vi "Main.vi"() -> ()   [LabVIEW 2015] (continued)
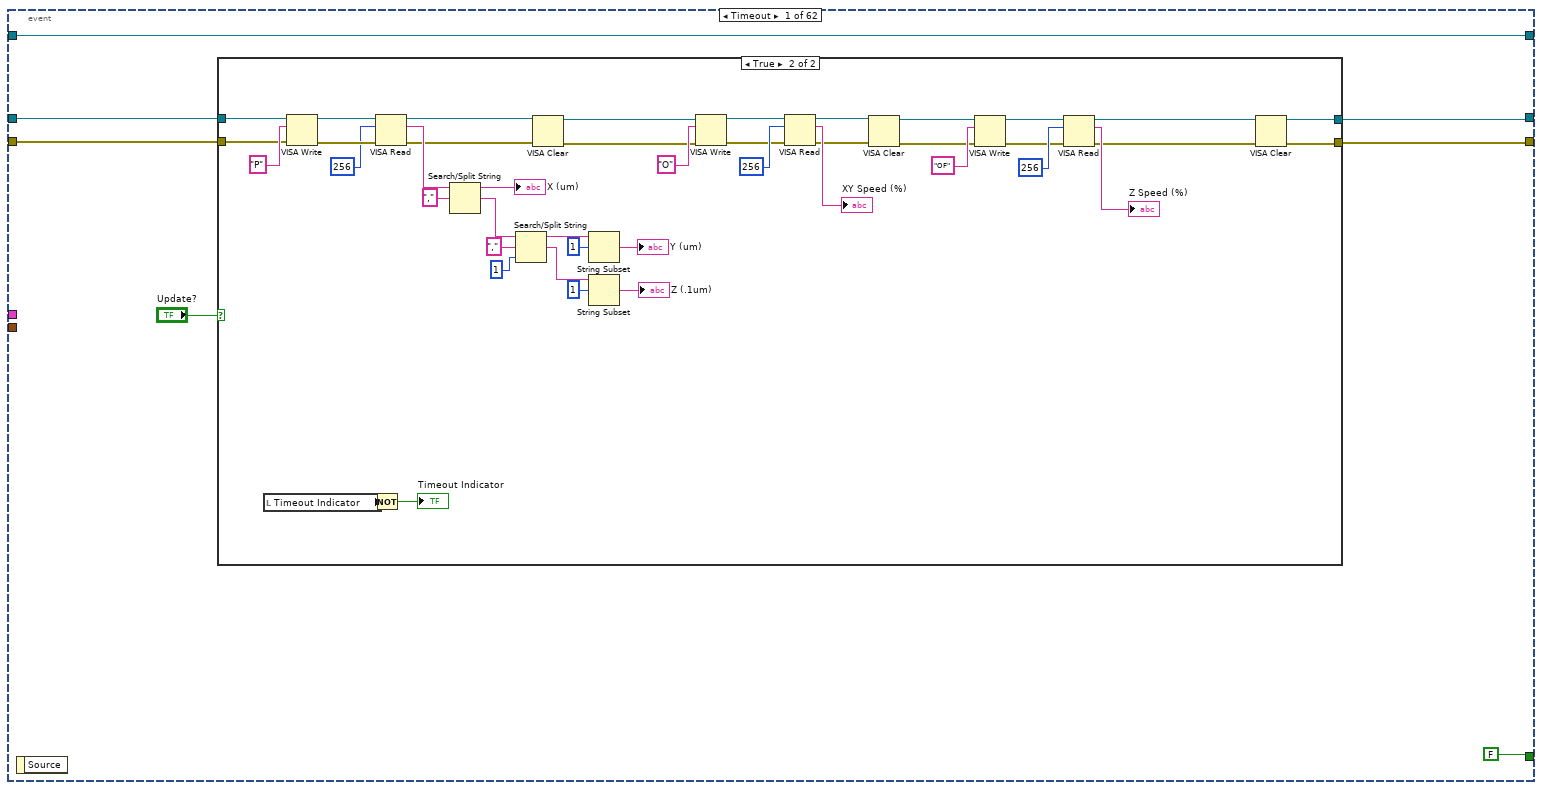
[diagram p3: hidden frame]
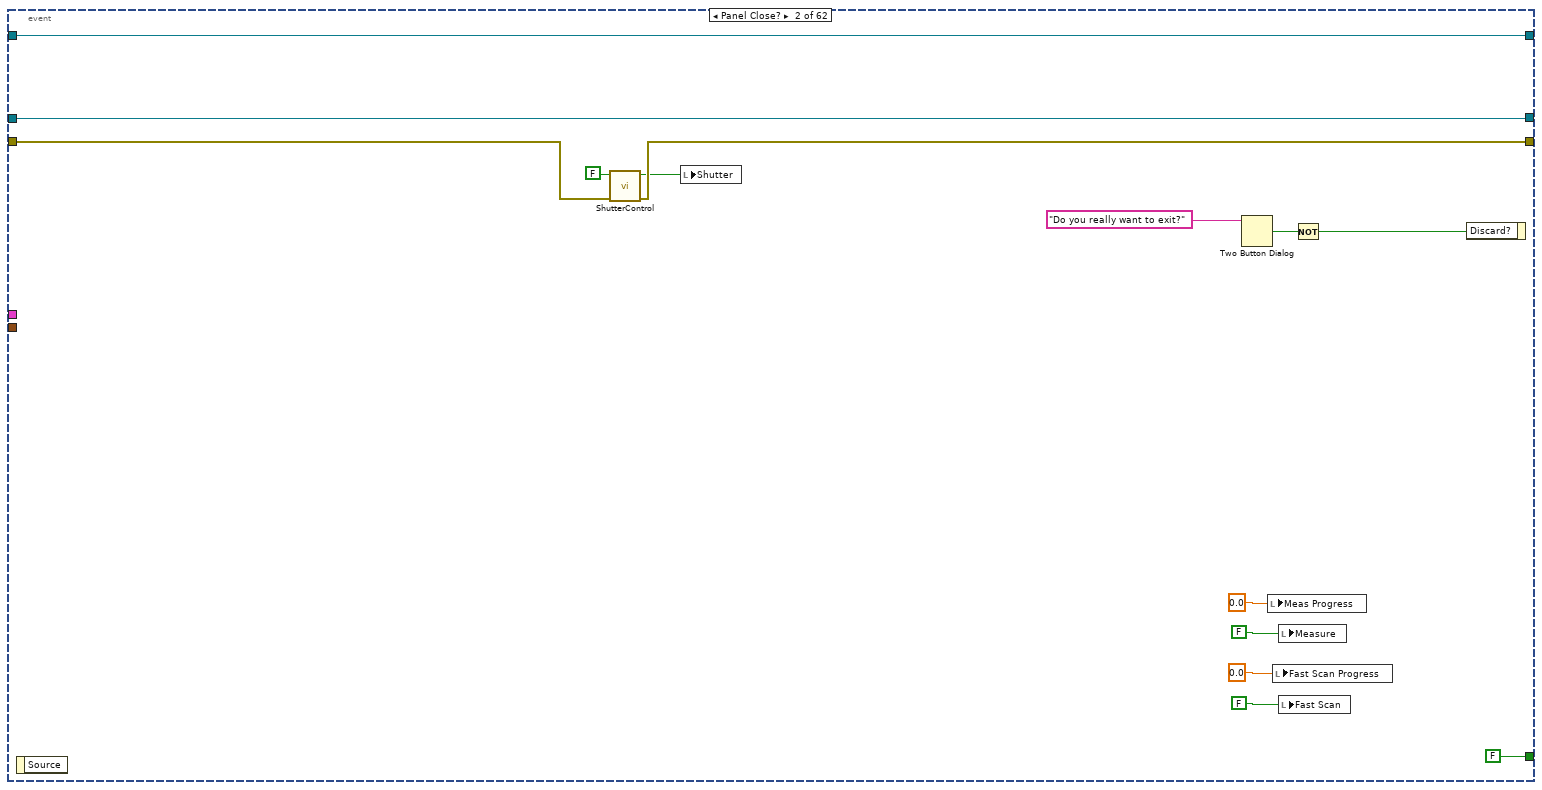
[diagram p5: hidden frame]
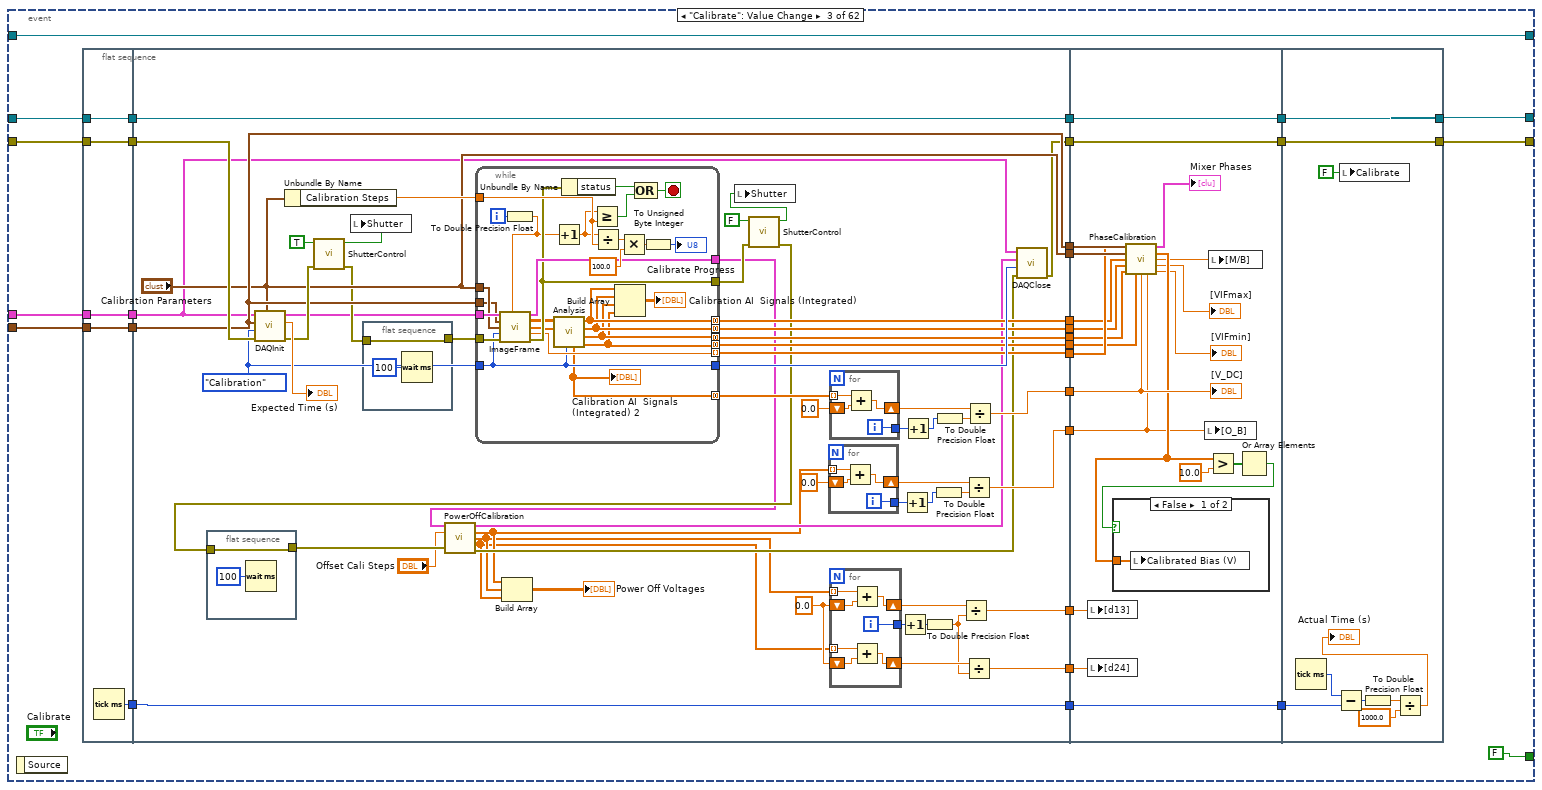
[diagram p6: hidden frame]
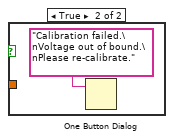
[diagram p7: hidden frame]
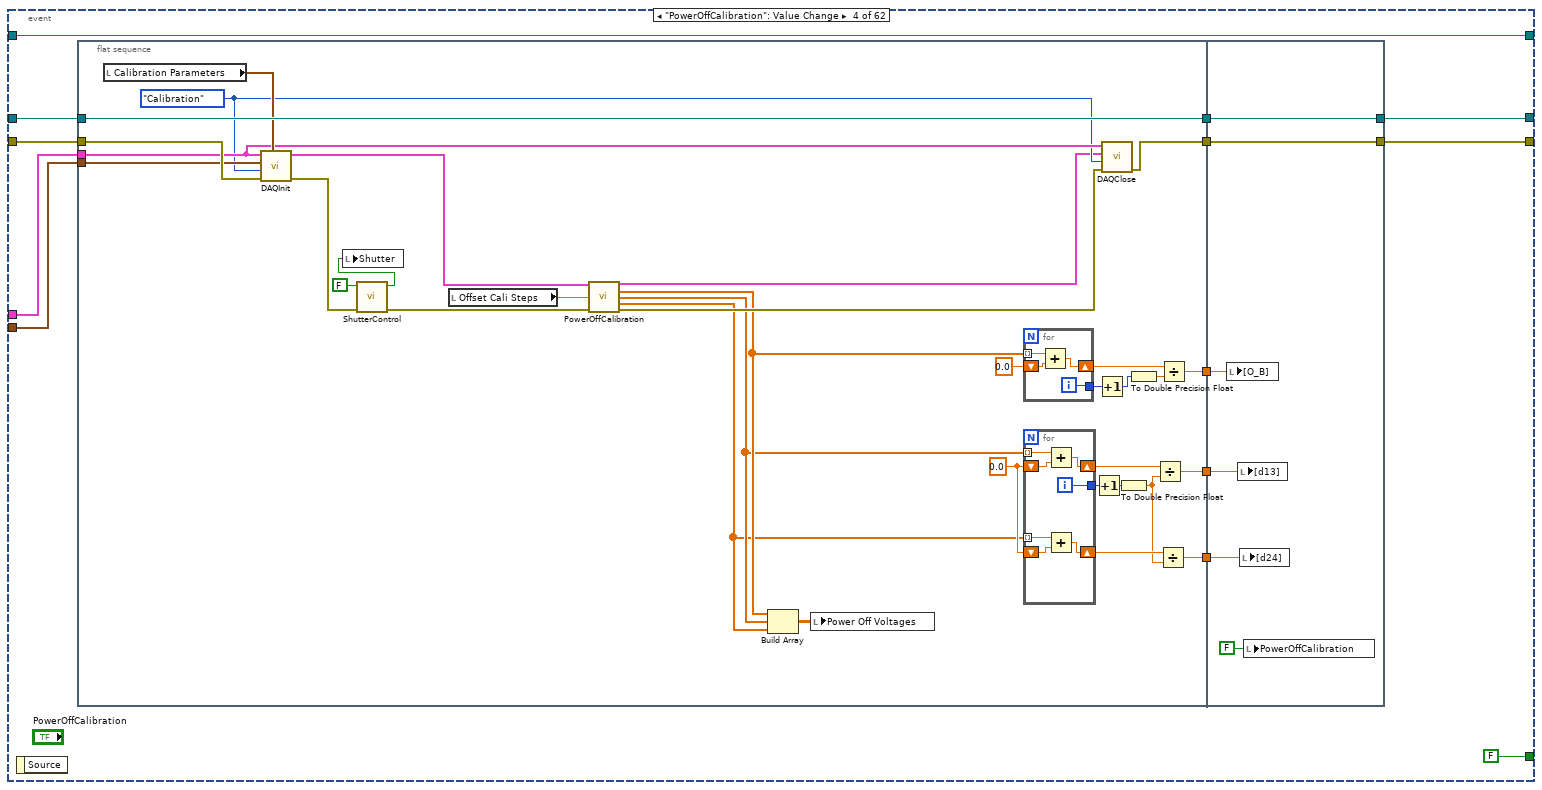
[diagram p8: hidden frame]
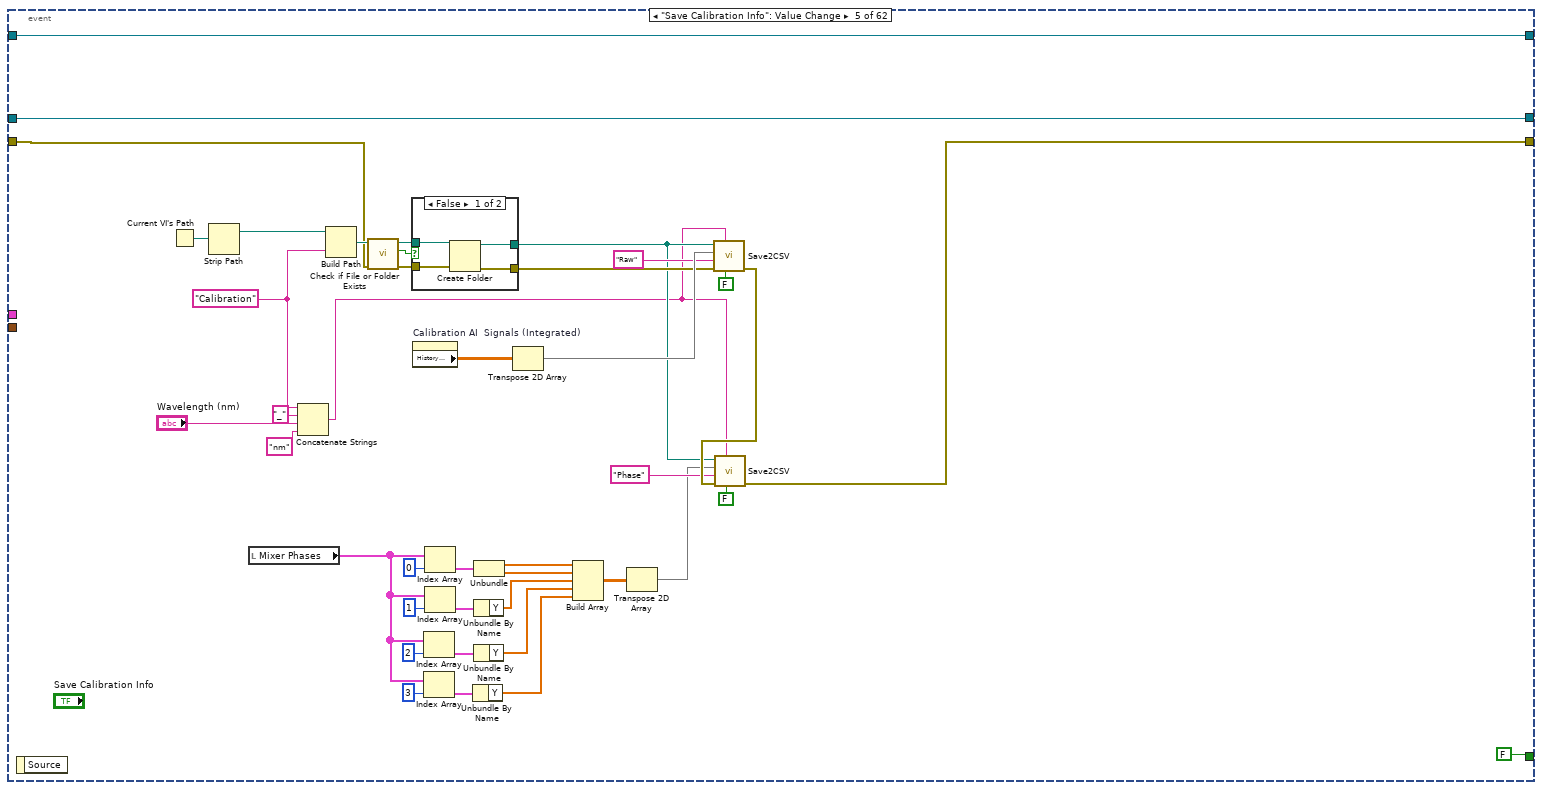
[diagram p9: hidden frame]
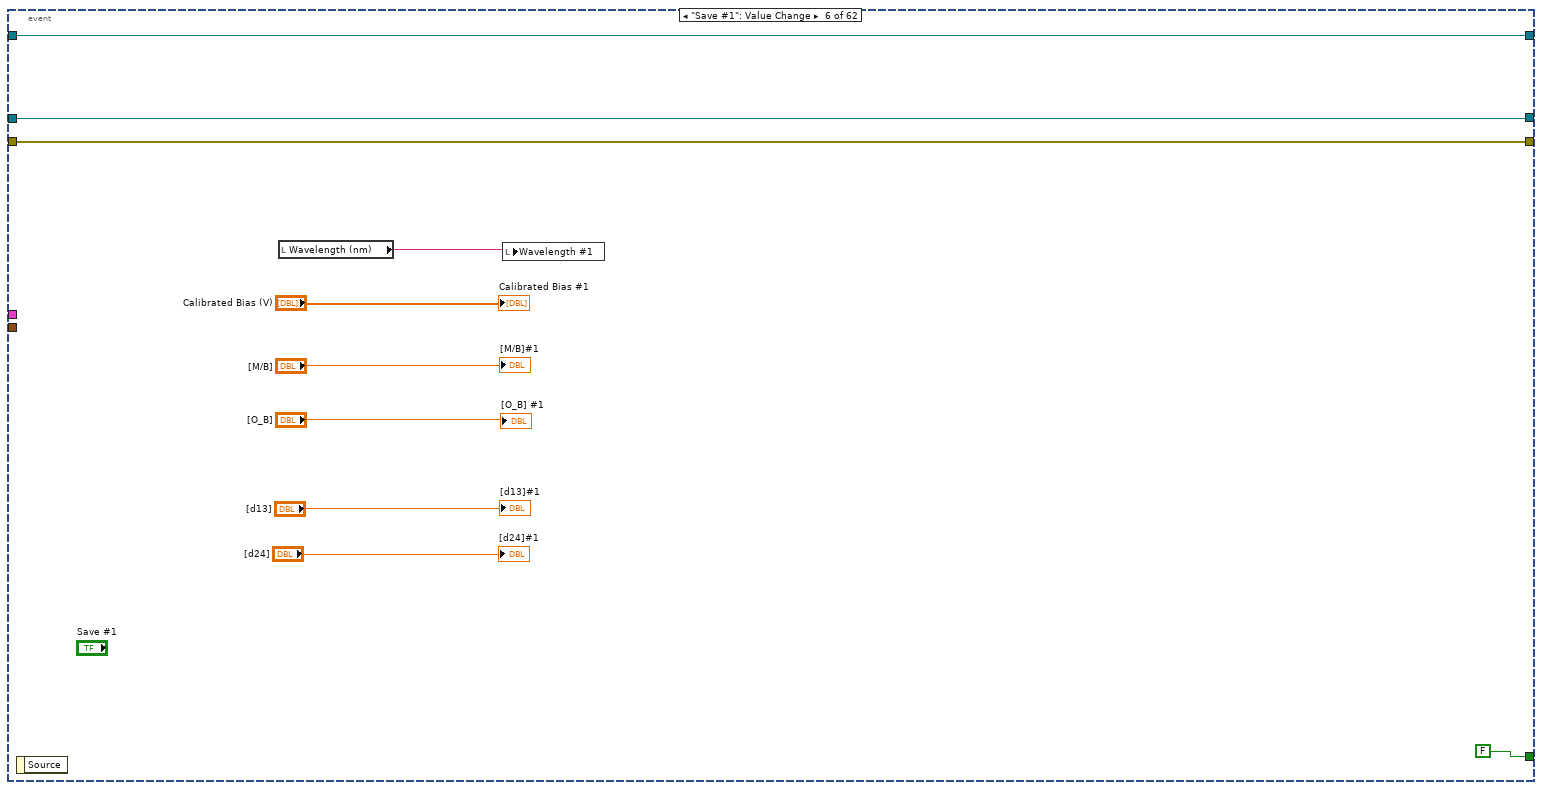
[diagram p11: hidden frame]
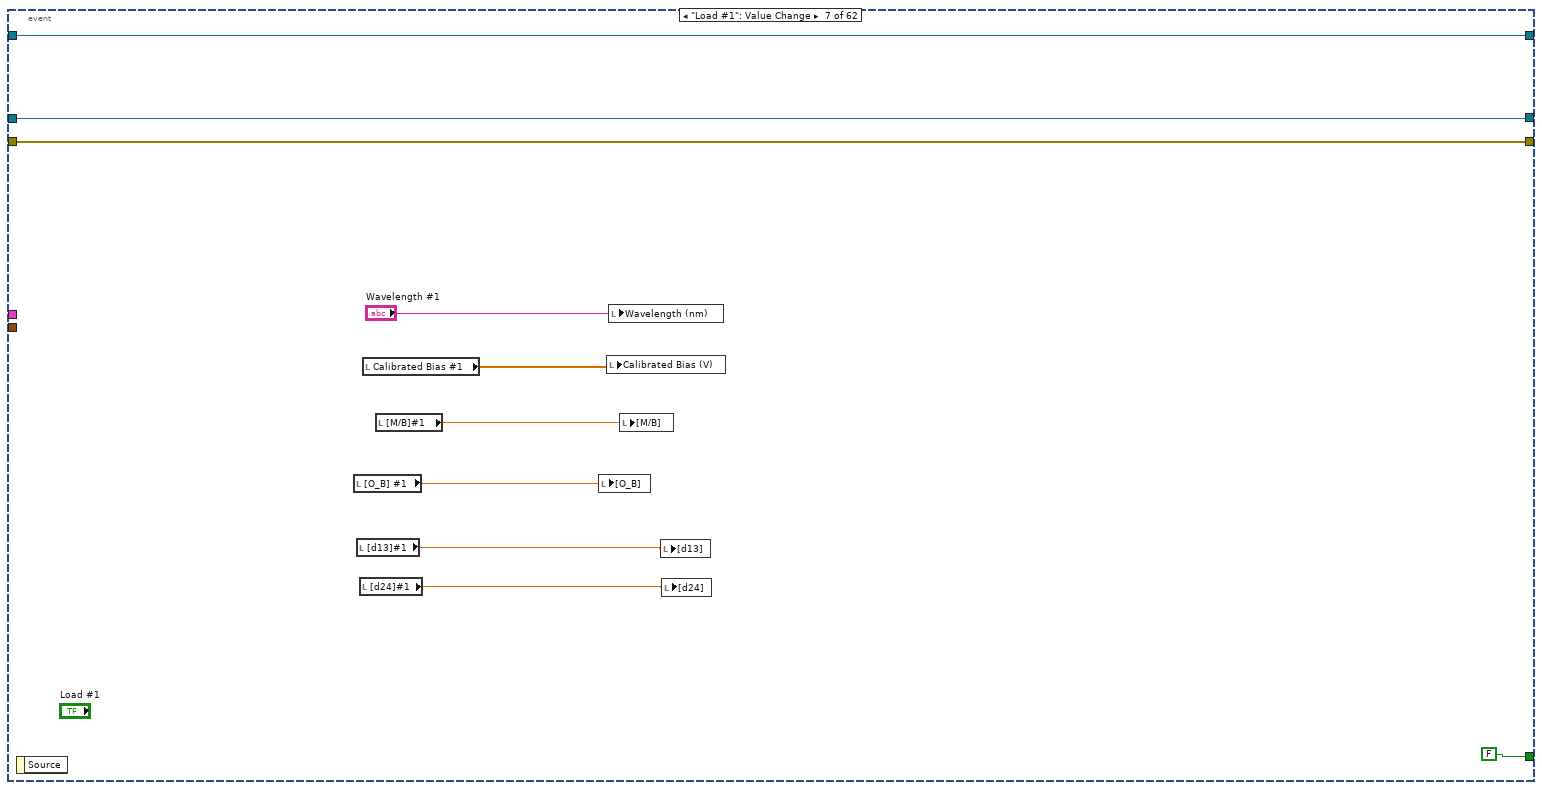
[diagram p12: hidden frame]
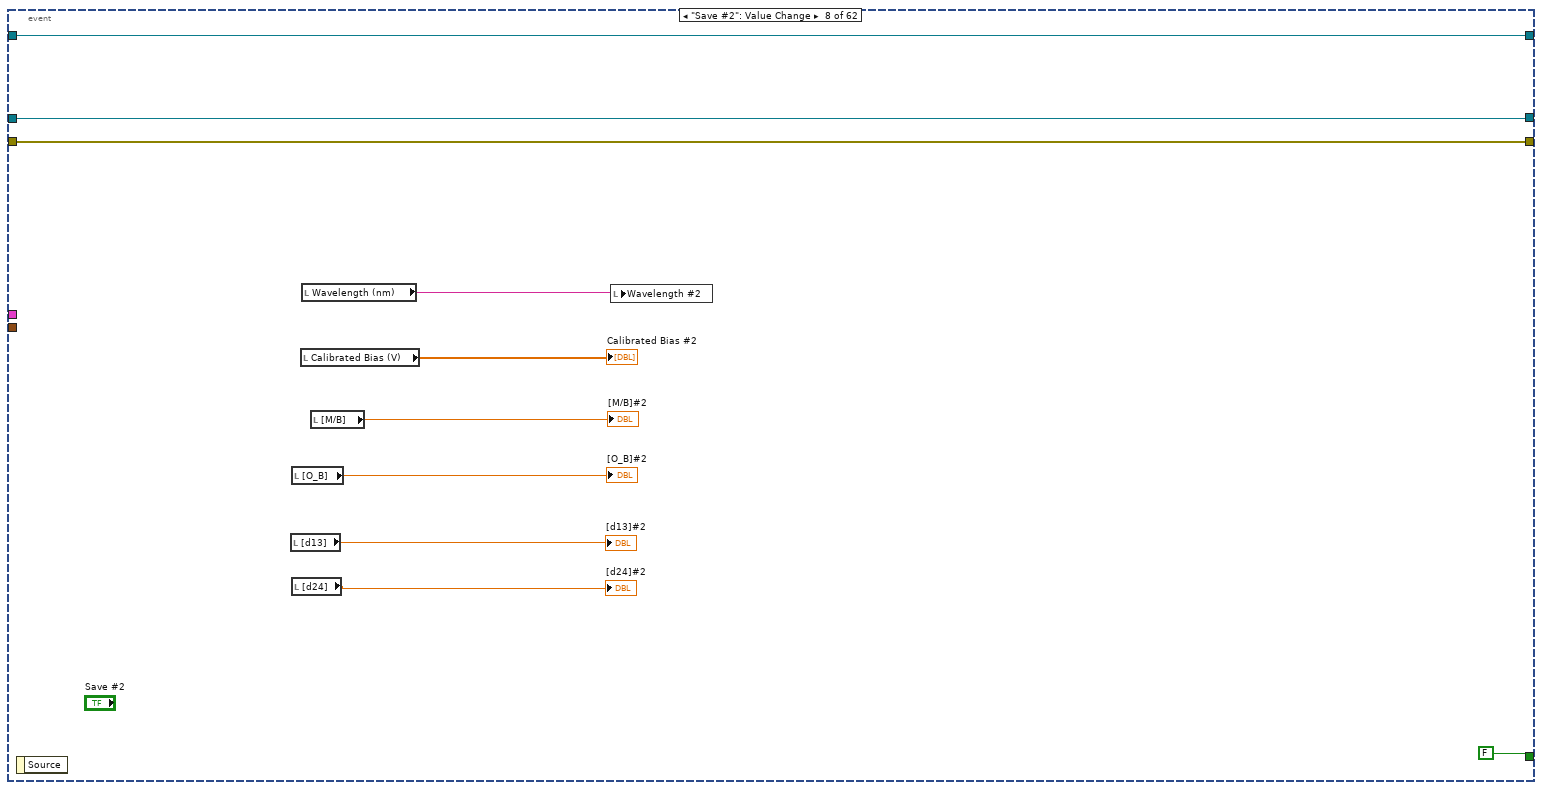
[diagram p13: hidden frame]
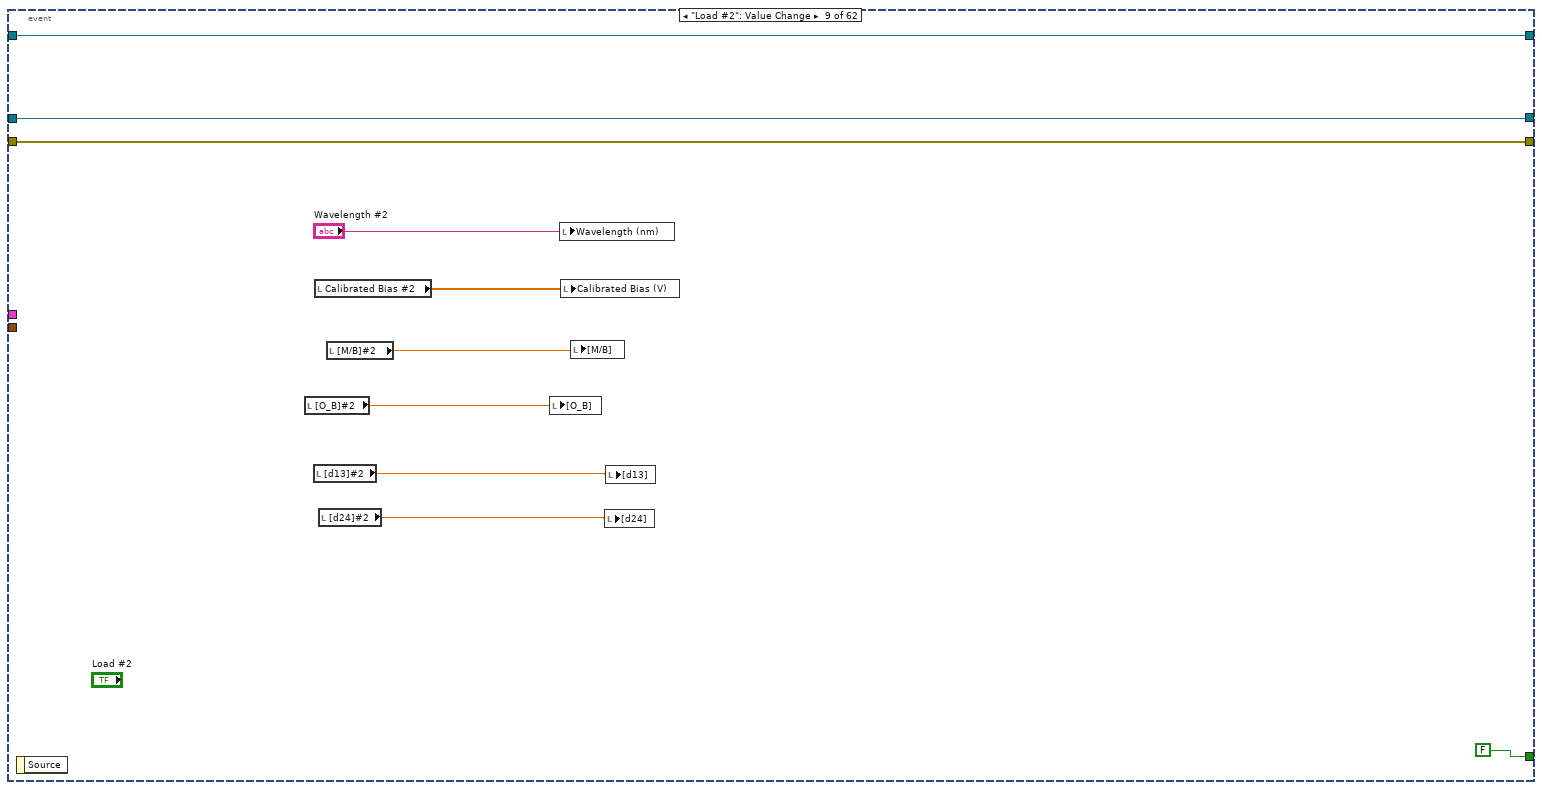
[diagram p14: hidden frame]
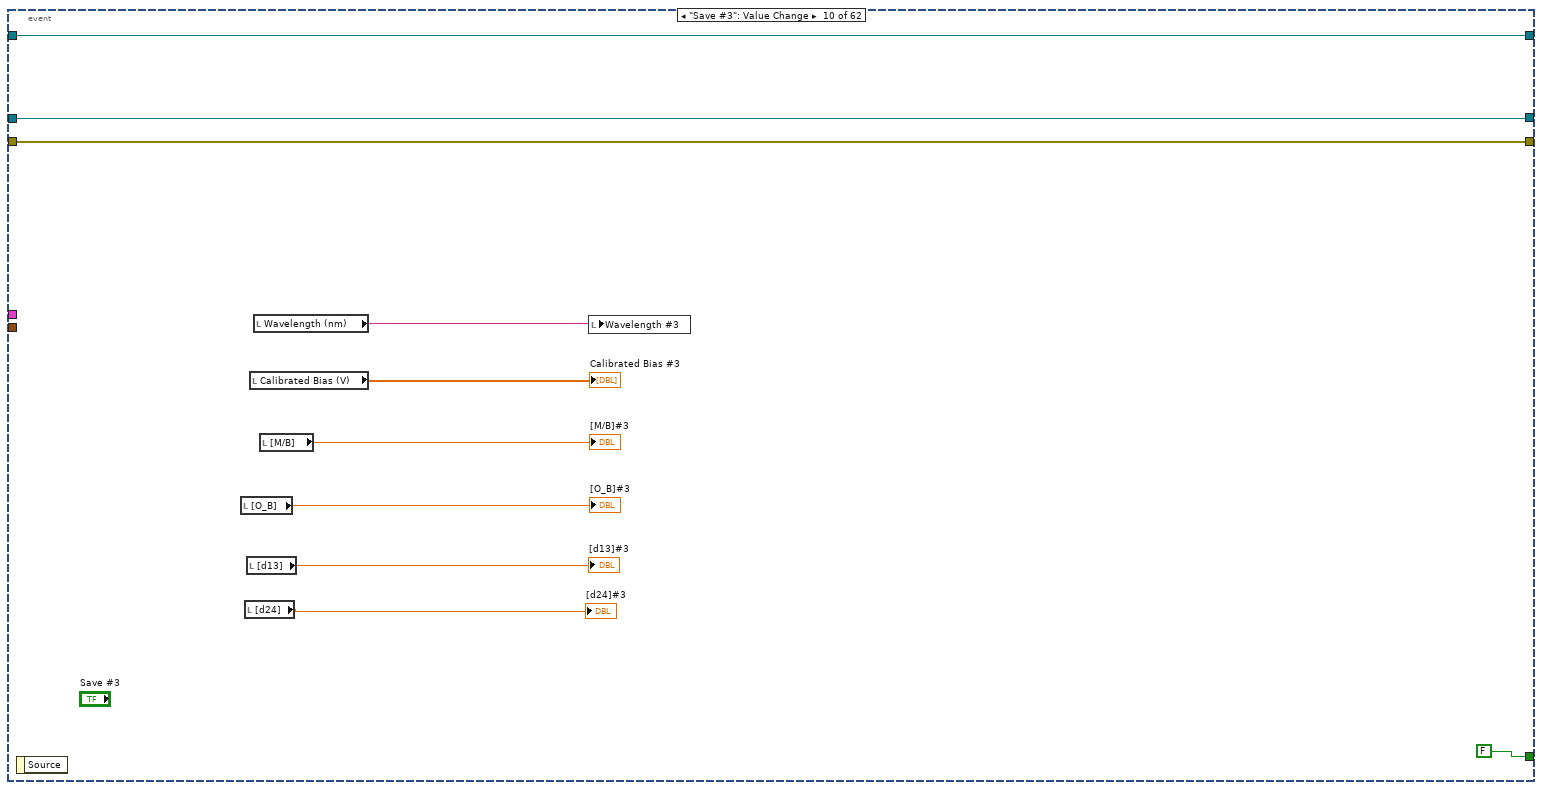
[diagram p15: hidden frame]
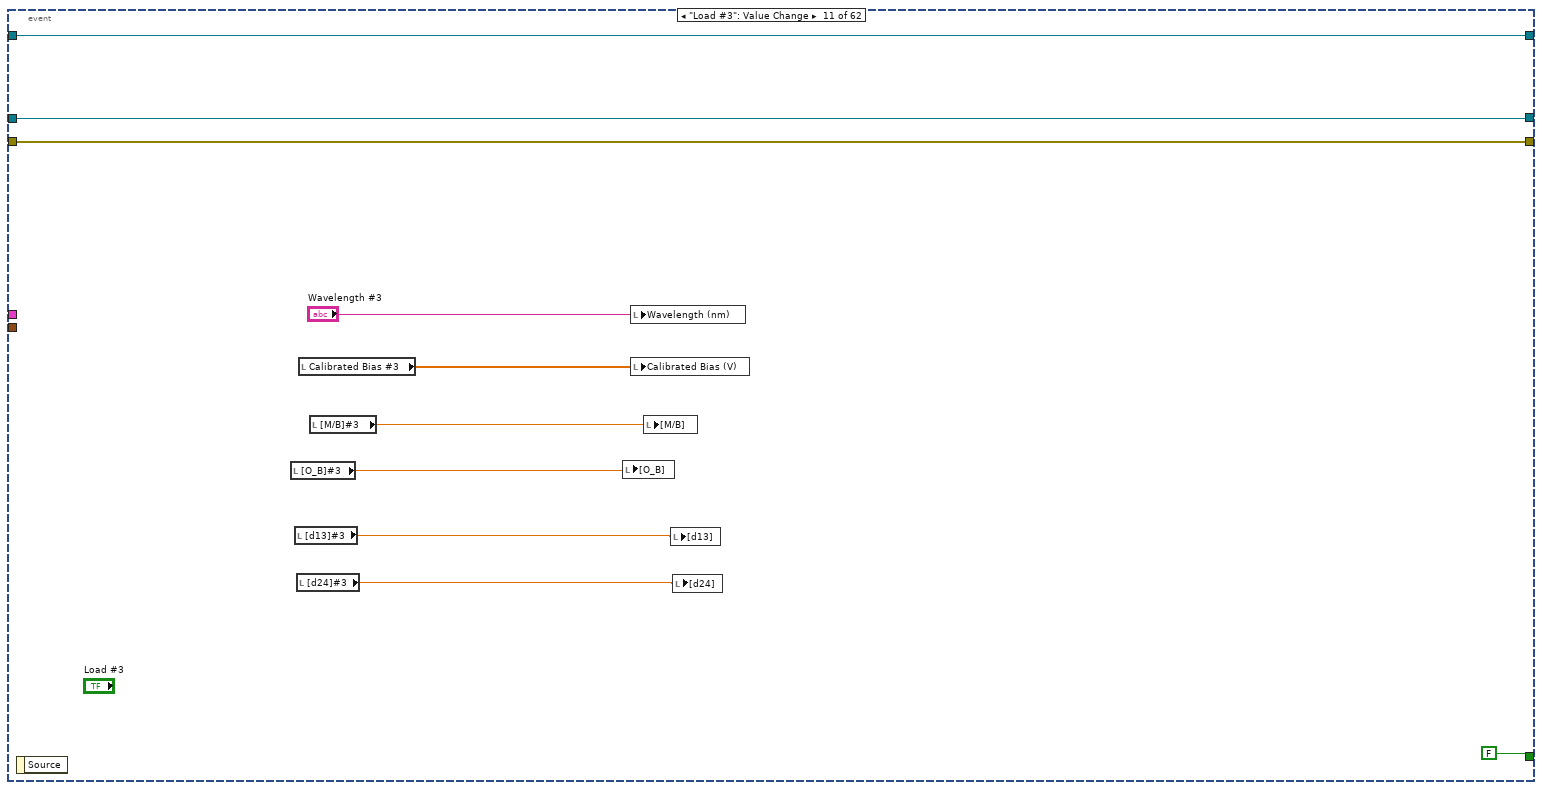
[diagram p16: hidden frame]
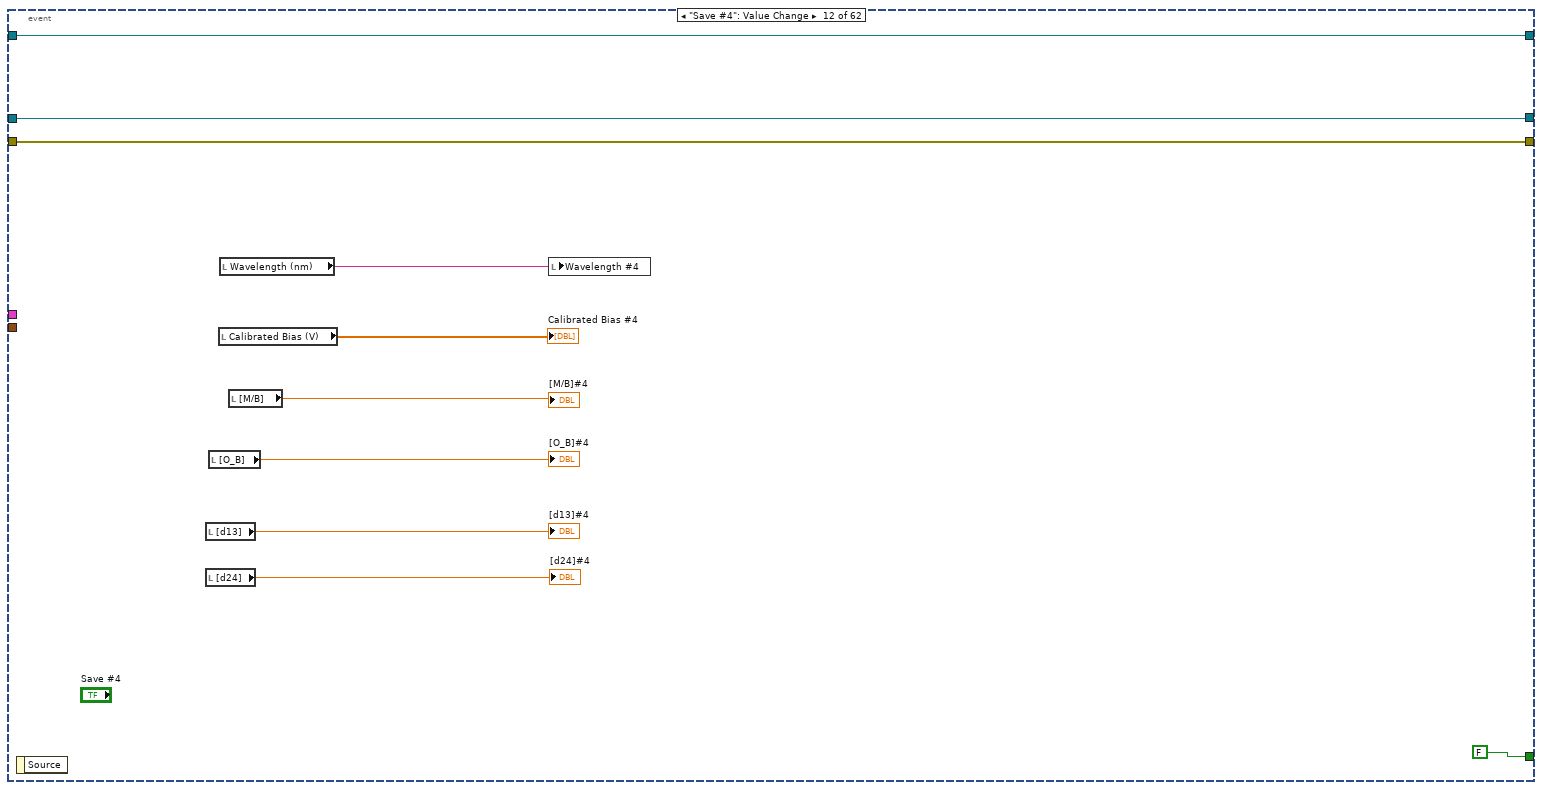
[diagram p17: hidden frame]
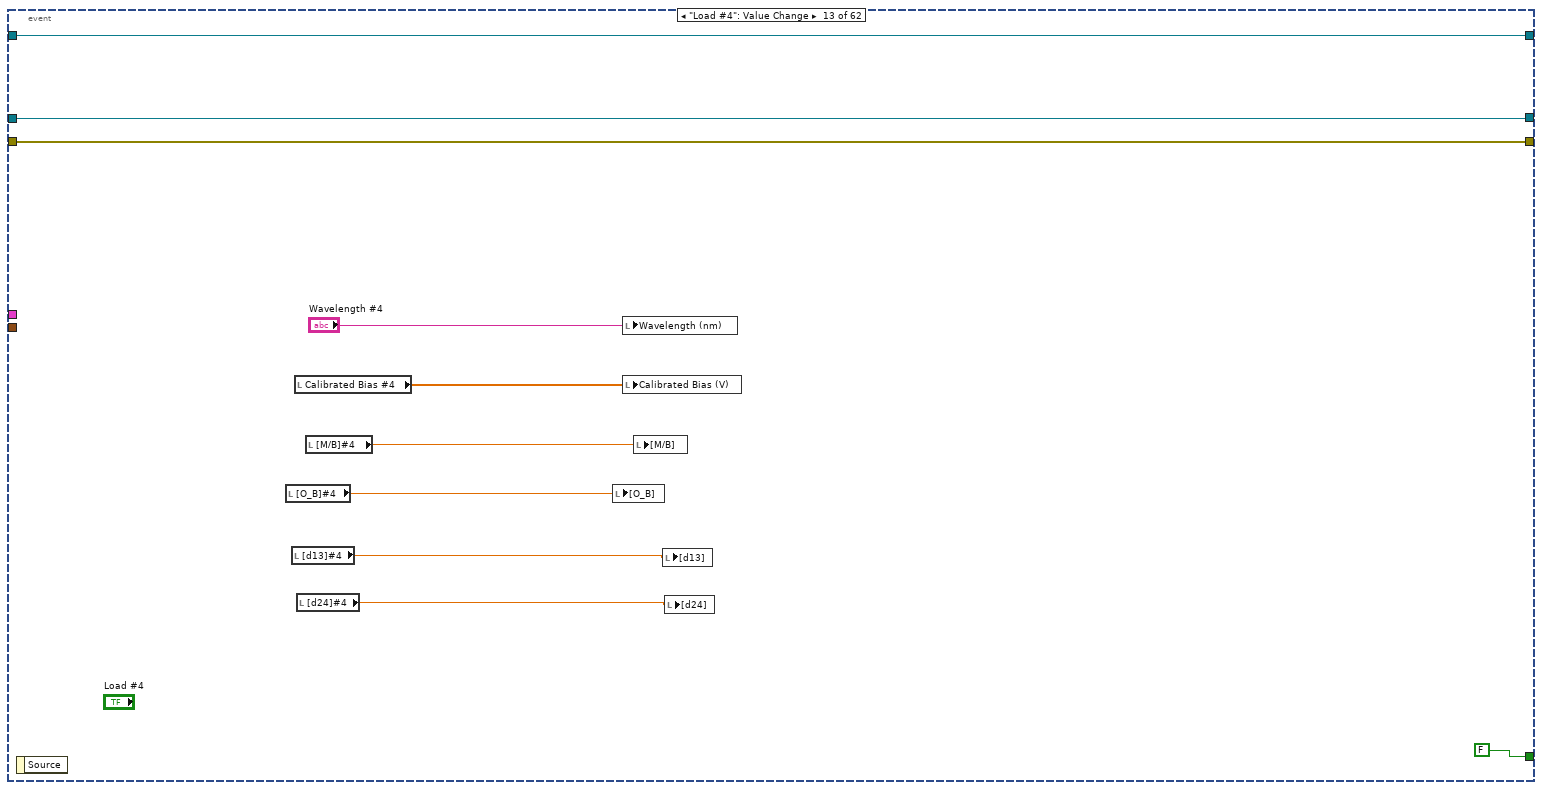
[diagram p18: hidden frame]
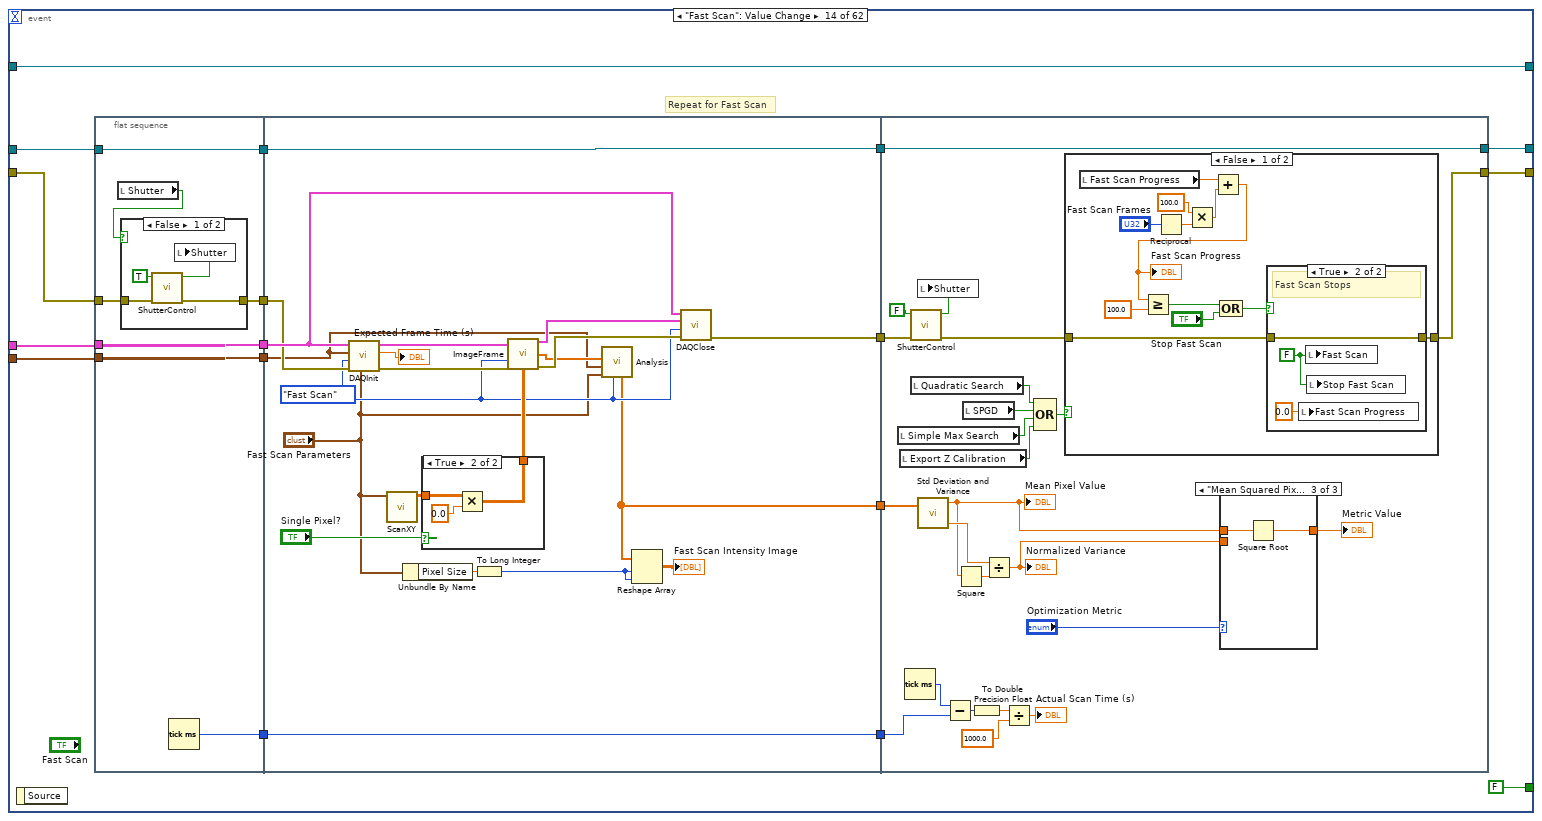
[diagram p19: hidden frame]
        n1435 = VISA Clear(VISA resource name=w2635, error in (no error)=w2638) -> (VISA resource name out=w2636:refnum<visa-resource-name>, error out=w2637:errorcluster)
      }
      event "Set Current Z to 0": Value Change {
        n1436 = event-data() -> ()  [unwired: 1 in, 1 out]
        n1437 = VISA Write(VISA resource name=w2652, write buffer="PZ,0" ("string"), error in (no error)=w2651) -> (VISA resource name out=w2654:refnum<visa-resource-name>, error out=w2653:errorcluster)  [unwired: 1 out]
        n1438 = VISA Read(VISA resource name=w2654, byte count=u32 256, error in (no error)=w2653) -> (VISA resource name out=w2647:refnum<visa-resource-name>, error out=w2650:errorcluster)  [unwired: 2 out]
        n1439 = VISA Clear(VISA resource name=w2647, error in (no error)=w2650) -> (VISA resource name out=w2648:refnum<visa-resource-name>, error out=w2649:errorcluster)
      }
      event "Report Position": Value Change {
        n1440 = event-data() -> ()  [unwired: 1 in, 1 out]
        n1441 = VISA Write(VISA resource name=w2684, write buffer="P" ("string"), error in (no error)=w2685) -> (VISA resource name out=w2691:refnum<visa-resource-name>, error out=w2690:errorcluster)  [unwired: 1 out]
        n1442 = VISA Read(VISA resource name=w2691, byte count=u32 256, error in (no error)=w2690) -> (VISA resource name out=w2667:refnum<visa-resource-name>, read buffer=w2696:string, error out=w2670:errorcluster)  [unwired: 1 out]
        n1443 = Search/Split String(string=w2696, search string/char (-)=",") -> (substring before match=w2683:string, match + rest of string=w2688:string)  [unwired: 1 in, 1 out]
        n1444 = Search/Split String(string=w2688, search string/char (-)=",", offset (0)=1) -> (substring before match=w2686:string, match + rest of string=w2697:string)  [unwired: 1 out]
        n1445 = local write "X (um)"(w2683) -> ()
        n1446 = String Subset(string=w2686, offset (0)=1) -> (substring=w2682:string)  [unwired: 1 in]
        n1447 = String Subset(string=w2697, offset (0)=1) -> (substring=w2681:string)  [unwired: 1 in]
        n1448 = VISA Clear(VISA resource name=w2667, error in (no error)=w2670) -> (VISA resource name out=w2668:refnum<visa-resource-name>, error out=w2669:errorcluster)
        n1449 = local write "Z (.1um)"(w2681) -> ()
        n1450 = local write "Y (um)"(w2682) -> ()
        n1451 = VISA Write(VISA resource name=w2668, write buffer="O" ("string"), error in (no error)=w2669) -> (VISA resource name out=w2678:refnum<visa-resource-name>, error out=w2679:errorcluster)  [unwired: 1 out]
        n1452 = VISA Read(VISA resource name=w2678, byte count=u32 256, error in (no error)=w2679) -> (VISA resource name out=w2666:refnum<visa-resource-name>, read buffer=w2672:string, error out=w2665:errorcluster)  [unwired: 1 out]
        n1453 = local write "XY Speed (%)"(w2672) -> ()
        n1454 = VISA Clear(VISA resource name=w2666, error in (no error)=w2665) -> (VISA resource name out=w2663:refnum<visa-resource-name>, error out=w2664:errorcluster)
        n1455 = VISA Write(VISA resource name=w2663, write buffer="OF" ("string"), error in (no error)=w2664) -> (VISA resource name out=w2674:refnum<visa-resource-name>, error out=w2675:errorcluster)  [unwired: 1 out]
        n1456 = VISA Read(VISA resource name=w2674, byte count=u32 256, error in (no error)=w2675) -> (VISA resource name out=w2662:refnum<visa-resource-name>, read buffer=w2671:string, error out=w2659:errorcluster)  [unwired: 1 out]
        n1457 = local write "Z Speed (%)"(w2671) -> ()
        n1458 = VISA Clear(VISA resource name=w2662, error in (no error)=w2659) -> (VISA resource name out=w2661:refnum<visa-resource-name>, error out=w2660:errorcluster)
      }
      event "Record X1": Value Change {
        n1459 = event-data() -> ()  [unwired: 1 in, 1 out]
        n1460 = property on="Fast Scan Intensity Image" class="IntGraph (strict)"(error in=w2702) -> (error out=w2701:errorcluster, "Cursor.Cursor X"=→"X1 (px)":dbl)  [unwired: 1 in, 1 out]
      }
      event "Record X2": Value Change {
        n1461 = event-data() -> ()  [unwired: 1 in, 1 out]
        n1462 = property on="Fast Scan Intensity Image" class="IntGraph (strict)"(error in=w2710) -> (error out=w2709:errorcluster, "Cursor.Cursor X"=→"X2 (px)":dbl)  [unwired: 1 in, 1 out]
      }
      event "Calculate Pixel Width": Value Change {
        n1463 = event-data() -> ()  [unwired: 1 in, 1 out]
        n1464 = local read "X2 (px)"() -> (w2716:dbl)
        n1465 = local read "X1 (px)"() -> (w2717:dbl)
        n1466 = Subtract(x=w2717, y=w2716) -> (x-y=w2718:dbl)
        n1467 = Absolute Value(x=w2718) -> (abs(x)=w2715:dbl)
        n1468 = Divide(x=30000.0, y=w2715) -> (x/y=→"dX (nm/px)":dbl)
      }
      event "Calculate XY Factor": Value Change {
        n1469 = event-data() -> ()  [unwired: 1 in, 1 out]
        n1470 = local read "Fast Scan Parameters"() -> (w2730:T4)
        n1471 = local read "dX (nm/px)"() -> (w2723:dbl)
        n1472 = Unbundle By Name(w2730) -> ("XY Factor (1/V)"=w2728:dbl)
        n1473 = Divide(x="Desired Pixel Width (nm)", y=w2723) -> (x/y=w2729:dbl)
        n1474 = Multiply(x=w2729, y=w2728) -> (x*y=→"New XY Factor":dbl)
      }
      event "Calculate XY Based on Objective": Value Change {
        # "XY Factor acquired at 400 pixel size, 300 nm pixel width"
        n1475 = event-data() -> ()  [unwired: 1 in, 1 out]
        n1476 = case shown="\"Nikon 40X NA 0.8 WD=3.5mm\", Default" "Objective Lens" {
          tunnel: [0.19061 ("x") 0.13615 ("x")] -> w2739
          frame "Nikon 40X NA 0.8 WD=3.5mm", Default {
          }
          frame "Olympus 25X NA 1.05 WD=2mm" {
          }
        }
        n1477 = local read "Fast Scan Parameters"() -> (w2742:T4)
        n1478 = local read "Desired Pixel Width (nm)"() -> (w2734:dbl)
        n1479 = Unbundle By Name(w2742) -> ("Pixel Size"=w2736:dbl)
        n1480 = Divide(x=w2736, y=400.0) -> (x/y=w2741:dbl)
        n1481 = Divide(x=w2734, y=300.0) -> (x/y=w2740:dbl)
        n1482 = Multiply(x=w2741, y=w2740) -> (x*y=w2738:dbl)
        n1483 = Multiply(x=w2739, y=w2738) -> (x*y=w2737:dbl)
        n1484 = local write "New XY Factor"(w2737) -> ()
      }
    }
  }
  n1485 = local read "Use DM?"() -> (w1:bool)
  n1486 = VISA Close(VISA resource name=w17, error in (no error)=w16) -> (error out=w4:errorcluster)
  n1487 = case shown="True" w1 {
    tunnel: w5 -> [_ w2751]
    tunnel: w4 -> [w2748 w2750]
    tunnel: [w2748 w2749] -> w3
    frame False {
    }
    frame True {
      n1488 = call "TLDFMX Close.vi"("error in (no error)"=w2750, "instrument handle"=w2751) -> ("error out"=w2749:errorcluster)  [unwired: 9 in]
    }
  }
  n1489 = call <vilib>:"Simple Error Handler.vi"("error in (no error)"=w3) -> ()  [unwired: 4 in, 5 out]
